vi "paraCfgEditor.vi"() -> ()   [LabVIEW 2010]
panel:
  out "View row details":string[](array[string])
  in  "Generate paraCfg.ini":bool
  in  "para section":string(tree)="parameter section"
  in  "Parameter CFG EDIT":string[][](table)
  out "error out":errorcluster
  in  "error in":errorcluster
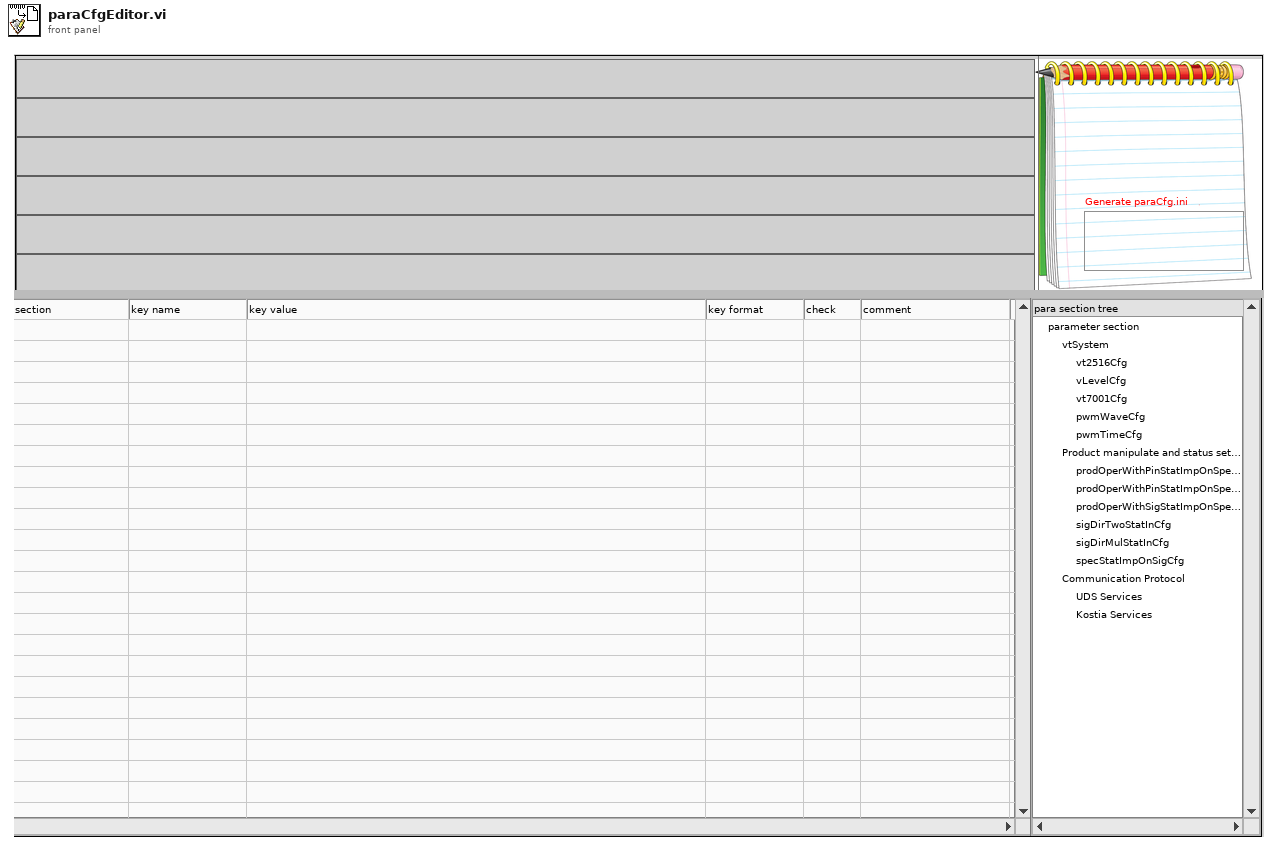
[diagram p1: front panel]
types:
  T1 = typedef "LVRowAndColumnTypeDef.ctl" = cluster{"Row":i32, "Column":i32}
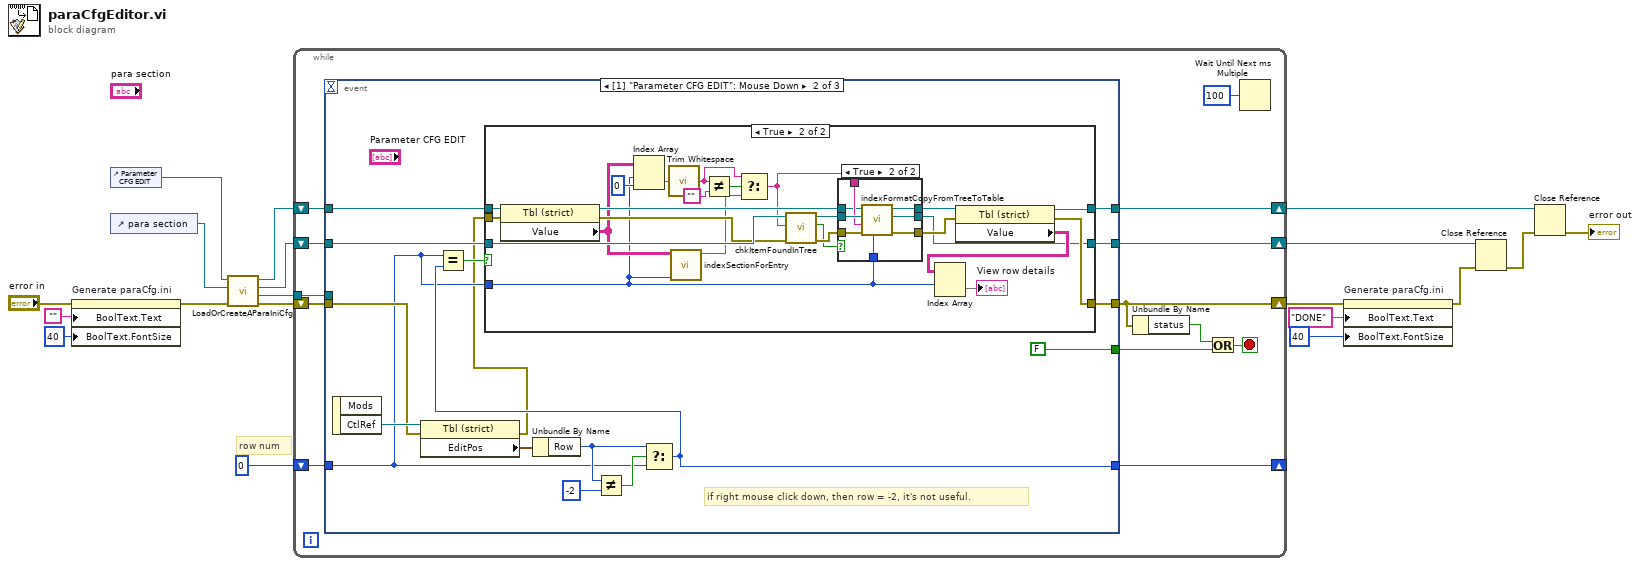
[diagram p0: block diagram]
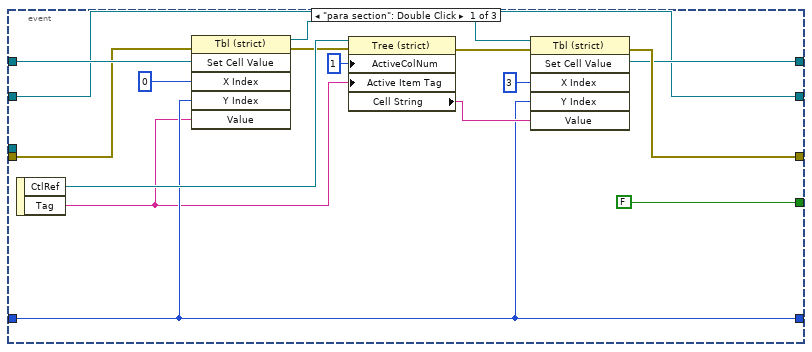
[diagram p2: hidden frame]
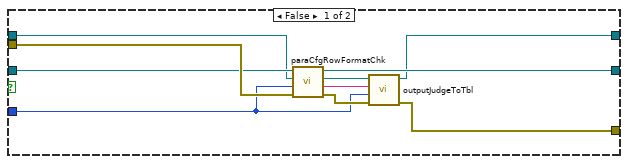
[diagram p3: hidden frame]
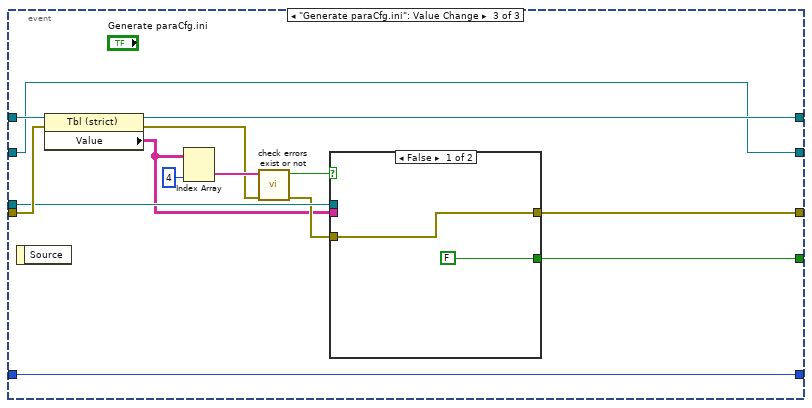
[diagram p5: hidden frame]
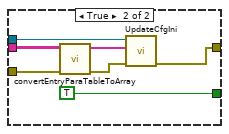
[diagram p6: hidden frame]
diagram:
  # "row num"
  n1 = property on="Generate paraCfg.ini" class="Bool"(error in="error in", "BoolText.Text"="", "BoolText.FontSize"=u32 40 ("Boolean Text.Font:Size")) -> (error out=w5:errorcluster)  [unwired: 1 in, 1 out]
  n2 = control-ref of="Parameter CFG EDIT"() -> (w10:refnum<vi>)
  n3 = control-ref of="para section"() -> (w9:refnum<vi>)
  n4 = call "LoadOrCreateAParaIniCfg.vi"("error in"=w5, "Tree Refnum"=w9, "Tbl Refnum in"=w10) -> ("error out"=w14:errorcluster, "cfg file refnum out"=w18:refnum<file>, "Tree Refnum out"=w13:refnum<vi>, "Tbl Refnum out"=w15:refnum<vi>)  [unwired: 5 in]
  n5 = while {
    shift-right: [w29] -> w4
    shift-left: w14 -> [w32]
    shift-right: [w25] -> _
    shift-left: 0 ("Row") -> [w26]
    shift-right: [w24] -> w17
    shift-left: w15 -> [w27]
    tunnel: w18 -> [w23]
    shift-right: [w21] -> w12
    shift-left: w13 -> [w22]
    stop <- w30 stop-if-true
    n6 = event shown="[1] \"Parameter CFG EDIT\": Mouse Down" {
      selector: _ -> [_ _ _]
      dyn-events: _ -> [_ _ _]
      timeout: _ -> [_ _ _]
      tunnel: w32 -> [w47 w55 w119]
      tunnel: [w38 w59 w120] -> w29
      tunnel: [FALSE ("stop") FALSE ("stop") w123] -> w31
      tunnel: w27 -> [w48 w52 w121]
      tunnel: w26 -> [w36 w50 w122]
      tunnel: [w36 w51 w122] -> w25
      tunnel: [w35 w57 w114] -> w24
      tunnel: w23 -> [_ _ w118]
      tunnel: w22 -> [w34 w54 w110]
      tunnel: [w34 w53 w110] -> w21
      event "para section": Double Click {
        n7 = event-data() -> ("CtlRef"=w45:refnum<vi>, "Tag"=w33:string)  [unwired: 1 in]
        n8 = invoke class="Tbl (strict)" method="Set Cell Value"(reference=w48, error in=w47, "X Index"=u32 0 ("Y Index"), "Y Index"=w36, "Value"=w33) -> (reference out=w39:refnum<vi>, error out=w40:errorcluster)  [unwired: 1 in, 4 out]
        n9 = property class="Tree (strict)"(reference=w45, error in=w40, "ActiveColNum"=1 ("Active Cell:Active Column Number"), "Active Item Tag"=w33) -> (error out=w43:errorcluster, "Cell String"=w42:string)  [unwired: 1 out]
        n10 = invoke class="Tbl (strict)" method="Set Cell Value"(reference=w39, error in=w43, "X Index"=u32 3, "Y Index"=w36, "Value"=w42) -> (reference out=w35:refnum<vi>, error out=w38:errorcluster)  [unwired: 1 in, 4 out]
      }
      event "Parameter CFG EDIT": Mouse Down {
        # "if right mouse click down, then row = -2, it's not useful."
        n11 = event-data() -> ("CtlRef"=w64:refnum<vi>)  [unwired: 1 in, 1 out]
        n12 = property class="Tbl (strict)"(reference=w64, error in=w55) -> (error out=w49:errorcluster, "EditPos"=w63:T1)  [unwired: 1 out]
        n13 = Unbundle By Name(w63) -> ("Row"=w60:i32)
        n14 = Not Equal?(x=w60, y=-2) -> (x != y?=w61:bool)
        n15 = Select(t=w60, s=w61, f=w50) -> (s? t:f=w51:i32)
        n16 = Equal?(x=w50, y=w51) -> (x = y?=w58:bool)
        n17 = case shown="True" w58 {
          tunnel: w50 -> [w66 w77]
          tunnel: w52 -> [w65 w87]
          tunnel: w49 -> [w74 w86]
          tunnel: [w67 w93] -> w59
          tunnel: [w68 w95] -> w57
          tunnel: w54 -> [w73 w91]
          tunnel: [w72 w92] -> w53
          frame False {
            n18 = call "paraCfgRowFormatChk.vi"("error in"=w74, "Row number"=w66, "Tbl Refnum in"=w65, "Tree Refnum in"=w73) -> ("error out"=w70:errorcluster, "chkRes"=w71:string, "Tbl Refnum out"=w69:refnum<vi>, "Tree Refnum out"=w72:refnum<vi>)  [unwired: 4 in]
            n19 = call "outputJudgeToTbl.vi"("error in"=w70, "rowNum"=w66, "judgeRes"=w71, "Tbl Refnum in"=w69) -> ("error out"=w67:errorcluster, "Tbl Refnum Out"=w68:refnum<vi>)  [unwired: 6 in]
          }
          frame True {
            n20 = property class="Tbl (strict)"(reference=w87, error in=w86) -> (reference out=w84:refnum<vi>, error out=w85:errorcluster, "Value"=w78:string[][])
            n21 = Index Array(array=w78, index (row)=w77, index (col)=0 ("disabled index (col)")) -> (element=w82:string)
            n22 = call <vilib>:"Trim Whitespace.vi"("string"=w82) -> ("trimmed string"=w79:string)  [unwired: 1 in]
            n23 = call "indexSectionForEntry.vi"("rowNum"=w77, "tbl"=w78) -> ("indexSection"=w76:string)  [unwired: 8 in, 1 out]
            n24 = Not Equal?(x=w79, y="") -> (x != y?=w80:bool)
            n25 = Select(t=w79, s=w80, f=w76) -> (s? t:f=w75:string)
            n26 = call "chkItemFoundInTree.vi"("error in"=w85, "searchItem"=w75, "Tree Refnum in"=w91) -> ("error out"=w89:errorcluster, "FoundInTree?"=w88:bool, "Tree Refnum out"=w90:refnum<vi>)  [unwired: 6 in]
            n27 = case shown="True" w88 {
              tunnel: [w101 w109] -> w97
              tunnel: [w99 w108] -> w96
              tunnel: w77 -> [_ w102]
              tunnel: [w100 w107] -> w92
              tunnel: w90 -> [w100 w106]
              tunnel: w89 -> [w99 w105]
              tunnel: w75 -> [_ w104]
              tunnel: w84 -> [w101 w103]
              frame False {
              }
              frame True {
                n28 = call "indexFormatCopyFromTreeToTable.vi"("rowNum"=w102, "error in"=w105, "searchItem"=w104, "Tree Refnum In"=w106, "Tbl Refnum in"=w103) -> ("error out"=w108:errorcluster, "Tree Refnum Out"=w107:refnum<vi>, "Tbl Refnum Out"=w109:refnum<vi>)  [unwired: 4 in]
              }
            }
            n29 = property class="Tbl (strict)"(reference=w97, error in=w96) -> (reference out=w95:refnum<vi>, error out=w93:errorcluster, "Value"=w94:string[][])
            n30 = Index Array(array=w94, index (row)=w77) -> (element=→"View row details":string[])  [unwired: 1 in]
          }
        }
      }
      event "Generate paraCfg.ini": Value Change {
        n31 = event-data() -> ()  [unwired: 1 in, 1 out]
        n32 = property class="Tbl (strict)"(reference=w121, error in=w119) -> (reference out=w114:refnum<vi>, error out=w115:errorcluster, "Value"=w111:string[][])
        n33 = Index Array(array=w111, index (col)=4 ("disabled index (col)")) -> (element=w116:string[])  [unwired: 1 in]
        n34 = call "check errors exist or not.vi"("error in"=w115, "judge column"=w116) -> ("error out"=w113:errorcluster, "Go on?"=w112:bool)  [unwired: 8 in]
        n35 = case shown="False" w112 {
          tunnel: [FALSE ("stop") TRUE ("stop")] -> w123
          tunnel: [w124 w131] -> w120
          tunnel: w118 -> [_ w126]
          tunnel: w113 -> [w124 w130]
          tunnel: w111 -> [_ w129]
          frame False {
          }
          frame True {
            n36 = call "convertEntryParaTableToArray.vi"("error in"=w130, "entryParaTbl"=w129) -> ("error out"=w128:errorcluster, "contArr"=w127:string[])  [unwired: 8 in]
            n37 = call "UpdateCfgIni.vi"("error in"=w128, "contentArray"=w127, "iniCfgRefnumIn"=w126) -> ("error out"=w131:errorcluster)  [unwired: 7 in, 1 out]
          }
        }
      }
    }
    n38 = Unbundle By Name(w29) -> ("status"=w28:bool)
    n39 = Or(x=w28, y=w31) -> (x .or. y?=w30:bool)
    n40 = Wait Until Next ms Multiple(millisecond multiple=u32 100) -> ()  [unwired: 1 out]
  }
  n41 = property on="Generate paraCfg.ini" class="Bool"(error in=w4, "BoolText.Text"="DONE" ("Boolean Text.Text"), "BoolText.FontSize"=u32 40 ("Boolean Text.Font:Size")) -> (error out=w1:errorcluster)  [unwired: 1 in, 1 out]
  n42 = Close Reference(reference=w12, error in (no error)=w1) -> (error out=w11:errorcluster)
  n43 = Close Reference(reference=w17, error in (no error)=w11) -> (error out=→"error out":errorcluster)
